vi "Main.vi"() -> ()   [LabVIEW 2020] (continued)
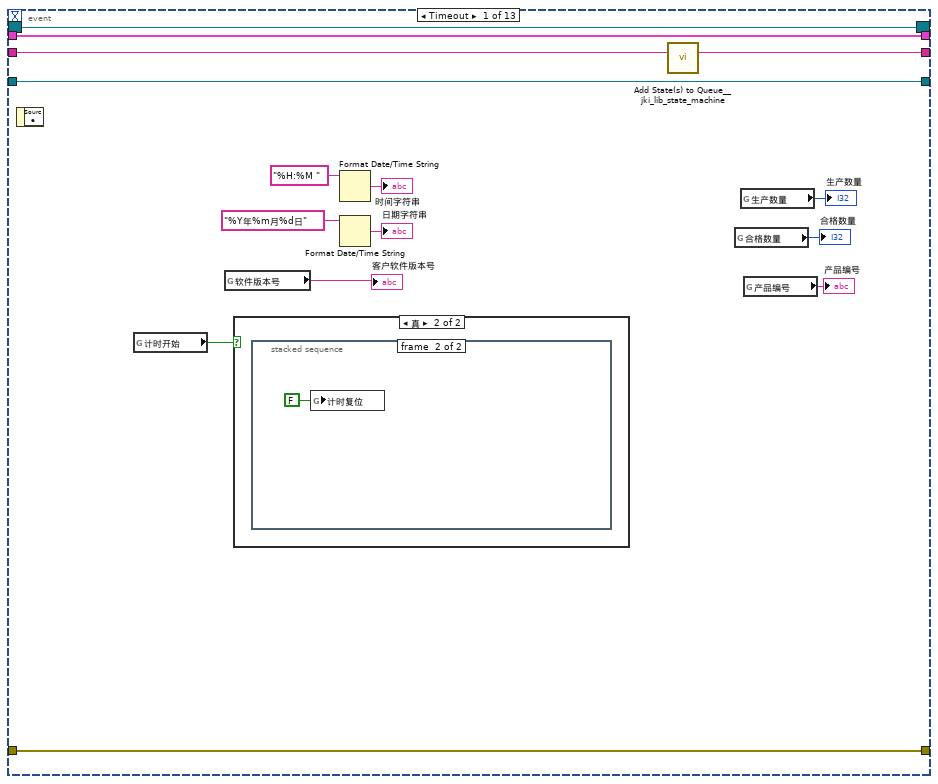
[diagram p2: hidden frame]
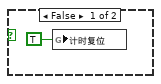
[diagram p3: hidden frame]
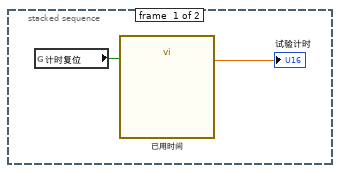
[diagram p4: hidden frame]
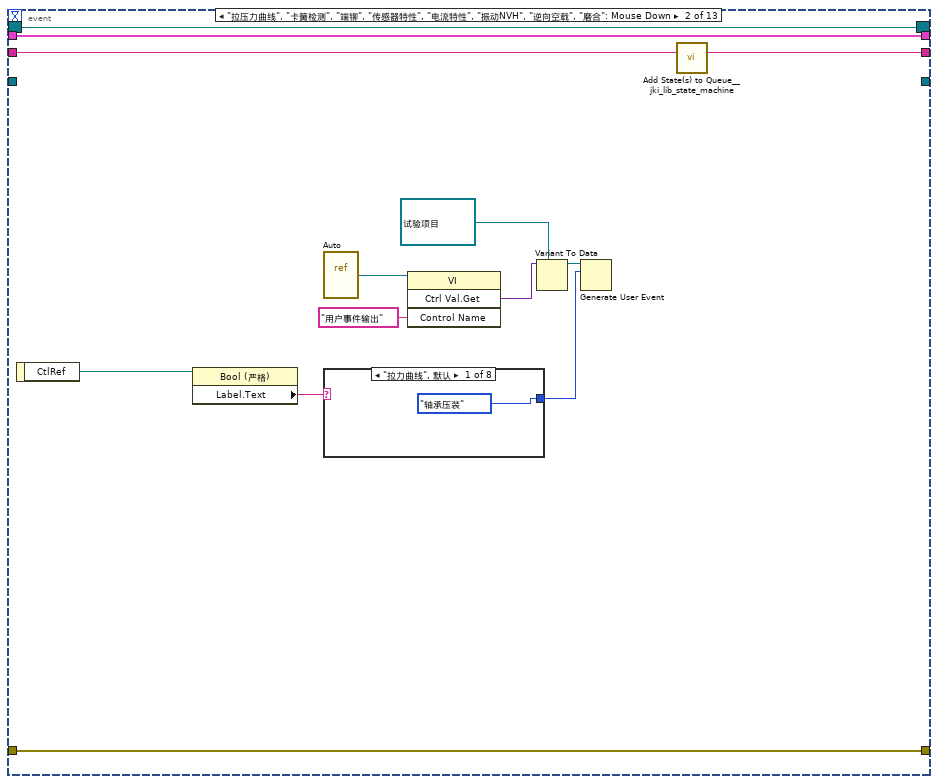
[diagram p5: hidden frame]
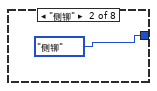
[diagram p6: hidden frame]
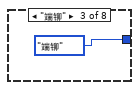
[diagram p7: hidden frame]
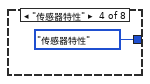
[diagram p8: hidden frame]
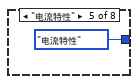
[diagram p9: hidden frame]
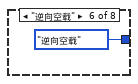
[diagram p10: hidden frame]
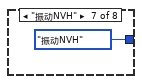
[diagram p11: hidden frame]
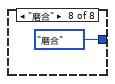
[diagram p12: hidden frame]
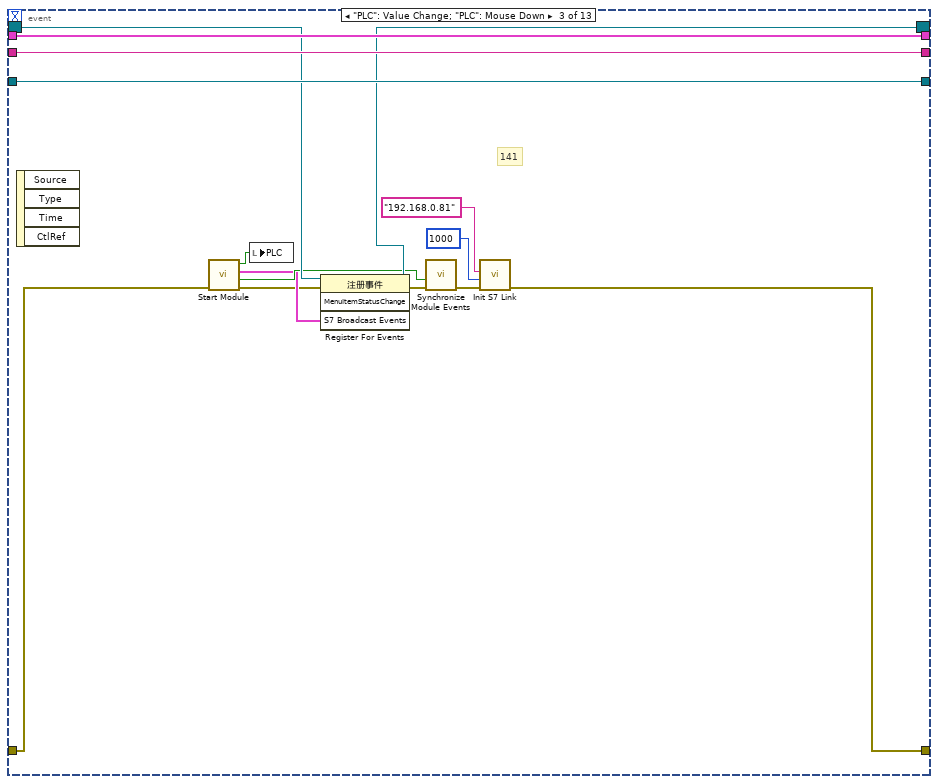
[diagram p13: hidden frame]
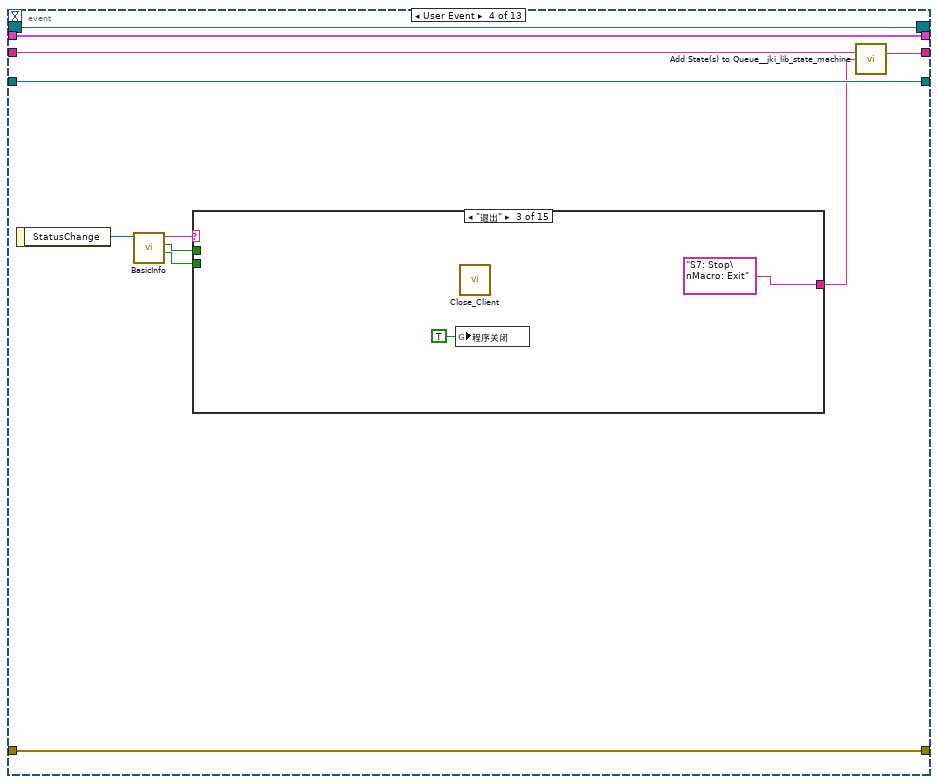
[diagram p14: hidden frame]
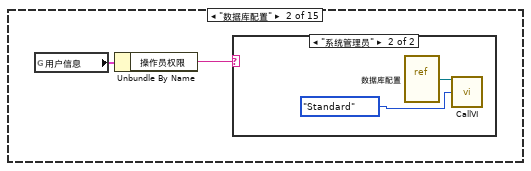
[diagram p16: hidden frame]
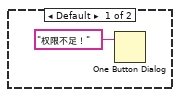
[diagram p17: hidden frame]
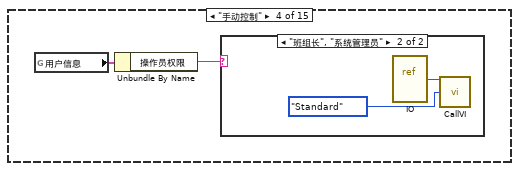
[diagram p18: hidden frame]
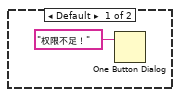
[diagram p19: hidden frame]
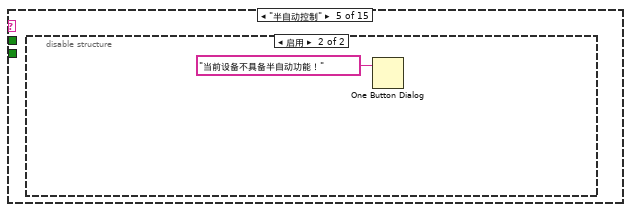
[diagram p20: hidden frame]
                    n120 = case shown="真" w200 {
                      frame False {
                      }
                      frame True {
                        n121 = vi-ref "Auto.vi"() -> (w204:refnum<vi>)
                        n122 = invoke class="VI" method="Ctrl Val.Set"(reference=w204, "Control Name"="STEP" ("控件名"), "Value"="退出自动" ("控件名")) -> ()  [unwired: 2 in, 5 out]
                      }
                    }
                  }
                }
              }
              frame Enabled {
              }
            }
            n123 = call <vilib>:"Add State(s) to Queue__jki_lib_state_machine.vi"("State(s) in (\"\")"=w190) -> ("States Out"=w191:string)  [unwired: 14 in]
          }
          event "错误": Mouse Down {
            n124 = event-data() -> ()  [unwired: 1 in, 8 out]
            n125 = vi-ref "报警信息.vi"() -> (w207:refnum<vi>)
            n126 = call "CallVI.vi"("VI引用"=w207, "状态"=T4."Standard") -> ()  [unwired: 12 in, 2 out]
            n127 = call <vilib>:"Add State(s) to Queue__jki_lib_state_machine.vi"("State(s) in (\"\")"=w209) -> ("States Out"=w210:string)  [unwired: 14 in]
          }
          event Panel Close? {
            n128 = event-data() -> ()  [unwired: 1 in, 1 out]
            n129 = global write "Global.vi" "程序关闭"(TRUE ("程序关闭")) -> ()
            n130 = call <vilib>:"Add State(s) to Queue__jki_lib_state_machine.vi"("State(s) in Front (\"\")"="S7: Stop\nMacro: Exit", "State(s) in (\"\")"=w219) -> ("States Out"=w218:string)  [unwired: 13 in]
            n131 = event-data("Discard?"=TRUE) -> ()  [unwired: 1 in, 1 out]
          }
          event "更换产品": Value Change {
            n132 = event-data() -> ("NewVal"=w221:refnum<vi>)  [unwired: 1 in, 5 out]
            n133 = stacked-sequence {
              tunnel: w221 -> [w226]
              frame #0 {
                n134 = stacked-sequence {
                  tunnel: w226 -> [w234 _]
                  frame #0 {
                    n135 = disable-structure shown="禁用" {
                      disable-tunnel: w234 -> [w236 _]
                      frame Disabled {
                        n136 = control-ref of="子面板"() -> (w235:refnum<vi>)
                        n137 = call "Call_SubPanal.vi"("VI引用句柄"=w236, "SubPnl引用句柄"=w235) -> ()  [unwired: 9 in, 1 out]
                      }
                      frame Enabled {
                      }
                    }
                    n138 = vi-ref "Auto.vi"() -> (w233:refnum<vi>)
                    n139 = invoke class="VI" method="Ctrl Val.Get"(reference=w233, "Control Name"="产品变更_Event" ("控件名")) -> ("Get Control Value Variant"=w231:variant)  [unwired: 2 in, 3 out]
                    n140 = global read "Global.vi" "产品型号"() -> (w228:string)
                    n141 = Variant To Data(type=refnum<user-event> refnum ("产品变更_Event"), Variant=w231) -> (data=w229:refnum<user-event>, error out=w227:errorcluster)  [unwired: 1 in]
                    n142 = Generate User Event(user event=w229, event data cluster=w228, error in=w227) -> ()  [unwired: 1 in, 2 out]
                    n143 = local write "产品型号"(w228) -> ()
                  }
                  frame #1 {
                    n144 = disable-structure shown="禁用" {
                      frame Disabled {
                        n145 = control-ref of="拉压力曲线"() -> (w238:refnum<vi>)
                        n146 = control-ref of="卡簧检测"() -> (w237:refnum<vi>)
                        n147 = global read "Global.vi" "试验项目"() -> (w241:bool[])
                        n148 = Build Array(w238, w237) -> (w240:refnum<vi>[])
                        n149 = for {
                          tunnel: w240 -> [w245] mode=indexing
                          tunnel: w241 -> [w246] mode=indexing
                          shift-right: [w242] -> _
                          shift-left: 2000 -> [w243]
                          i -> [w244]
                          n150 = case shown="真" w246 {
                            tunnel: w245 -> [w247 w255]
                            tunnel: w244 -> [_ _]
                            tunnel: w243 -> [w249 w252]
                            tunnel: [w249 w250] -> w242
                            frame False {
                              n151 = property class="Bool (严格)"(reference=w247, "Top"=2000) -> ()  [unwired: 1 in, 2 out]
                            }
                            frame True {
                              n152 = Add(x=w252, y=135) -> (x+y=w250:i32)
                              n153 = Bundle(w250, 1235) -> (w253:cluster{i32, i32})  [unwired: 1 in]
                              n154 = property class="Bool (严格)"(reference=w255, "Position"=w253) -> ()  [unwired: 1 in, 2 out]
                            }
                          }
                        }
                      }
                      frame Enabled {
                      }
                    }
                  }
                }
              }
            }
            n155 = call <vilib>:"Add State(s) to Queue__jki_lib_state_machine.vi"("State(s) in (\"\")"=w222) -> ("States Out"=w223:string)  [unwired: 14 in]
          }
          event "Andon": Value Change {
            n156 = event-data() -> ("NewVal"=w260:enum32{"未选择", "缺料报警", "质量报警", "故障报警"})  [unwired: 1 in]
            n157 = case shown="\"未选择\", 默认" w260 {
              tunnel: [enum16{"设备离线", "设备正常", "设备缺料", "设备故障", "质量报警"}."设备正常" ("设备状态") enum16{"设备离线", "设备正常", "设备缺料", "设备故障", "质量报警"}."设备缺料" ("设备状态") enum16{"设备离线", "设备正常", "设备缺料", "设备故障", "质量报警"}."质量报警" ("设备状态") enum16{"设备离线", "设备正常", "设备缺料", "设备故障", "质量报警"}."设备故障" ("设备状态")] -> w258
              frame "未选择", Default {
              }
              frame "缺料报警" {
              }
              frame "质量报警" {
              }
              frame "故障报警" {
              }
            }
            n158 = local read "userName"() -> (w257:string)
            n159 = Bundle By Name(cluster=T5 {"设备名称"="滑移力检测", "操作人员"="", "设备状态"=enum."设备离线", "附加信息"=""} ("设备信息"), "操作人员"=w257, "设备状态"=w258) -> (w256:T5)
            n160 = call "Change_Client.vi"("设备信息"=w256) -> ()  [unwired: 10 in, 1 out]
          }
        }
      }
      frame "---------- Core ----------" {
        n161 = call <vilib>:"Add State(s) to Queue__jki_lib_state_machine.vi"("State(s) in (\"\")"=w274) -> ("States Out"=w273:string)  [unwired: 14 in]
      }
      frame Default {
        w286 = 42 items=["No error", "Argument error", "Memory is full", "Out of zone", "End of file", "File already open", "Generic file I/O error", "File not found", "File permission error", "Disk is full", "Duplicate path", "Too many files open", "System feature not enabled", "Resource file not found", "Cannot add resource", "Resource not found", "Image not found", "Image memory error", "Pen does not exist", "Config type invalid", "Config token not found", "Config parse error", "Config memory error", "Bad external code format", "Bad external code offset", "External code not present", "Null window", "Destroy window error", "Null menu", "Print aborted", "Bad print record", "Print driver error", "Windows error during printing", "Memory error during printing", "Print dialog error", "Generic print error", "Invalid device refnum", "Device not found", "Device parameter error", "Device unit error", "Cannot open device", "Device call aborted", "Generic error", "Cancelled by user", "Object ID too low", "Object ID too high", "Object not in heap", "Unknown heap", "Unknown object (invalid DefProc)", "Unknown object (DefProc not in table)", "Message out of range", "Invalid (null) method", "Unknown message", "Manager call not supported", "Bad address", "Network operation in progress", "Network operation timed out", "Connection is busy", "Network attribute not supported", "Network error", "Address in use", "System out of memory", "Connection aborted", "Connection refused", "Not connected", "Already connected", "Connection closed", "Initialization error (interapplication manager)", "Bad occurrence", "Wait on unbound occurrence handler", "Occurrence queue overflow", "Datalog type conflict", "Unused", "Unrecognized type (interapplication manager)", "Memory corrupt", "Failed to make temporary DLL", "Old CIN version", "Drag socket not found", "Failed to load drop-object", "Failed to register OLE object", "Failed to release OLE object", "Format specifier type mismatch", "Unknown format specifier", "Too few format specifiers", "Too many format specifiers", "Scan failed", "Newer CIN version", "Error converting to variant", "Runtime menu error", "Password tampered", "Variant attribute not found", "Incompatible variant data type", "Event data is not available", "Event Store is not present", "Occurrence is not found", "Event Queue is not created", "Event info is not available", "Refnum passed is NULL", "Error retrieving Class GUID", "Error retrieving CoClass GUID", "Error retrieving TypeLib GUID.", "Bad built application magic bytes.", "Specific driver is different from the specific driver associated with the Logical Name.", "There is no session opened to the class driver.", "Max Error", "MAX - Error with config objects", "MAX - Error loading configuration", "MAX - Group not supported"]
        # "Current State"
        n162 = Format Into String(format string="Software Exception: Unhandled State \"%s\"." ("message"), error in=w282, w277) -> (resulting string=w285:string, error out=w284:errorcluster)  [unwired: 1 in]
        n163 = call <vilib>:"Error Cluster From Error Code.vi"("show call chain? (False)"=TRUE, "error in (no error)"=w284, "error message (\"\")"=w285, "error code (0)"=w286) -> ("error out"=w283:errorcluster)  [unwired: 5 in]
        n164 = call <vilib>:"Add State(s) to Queue__jki_lib_state_machine.vi"("State(s) in (\"\")"=w281) -> ("States Out"=w280:string)  [unwired: 14 in]
      }
      frame "Initialize Core Data" {
        # "originally closed?"
        # "exe?"
        n165 = property class="VI"() -> ("Front Panel.Open"=w297:bool)  [unwired: 2 in, 2 out]
        n166 = property class="App"() -> ("App.Kind"=w296:T6)  [unwired: 2 in, 2 out]
        n167 = control-ref of="Current VI Reference"() -> (w290:refnum<vi>)
        n168 = Not(x=w297) -> (.not. x?=w294:bool)
        n169 = Equal?(x=w296, y=T6."Run Time System" ("Application:Kind")) -> (x = y?=w293:bool)
        n170 = Or(x=w294, y=w293) -> (x .or. y?=w291:bool)
        n171 = Bundle By Name(cluster=w292, "Core.Current VI Reference"=w290, "Core.Close Panel on Exit?"=w291) -> (w299:T8)
        n172 = call <vilib>:"Add State(s) to Queue__jki_lib_state_machine.vi"("State(s) in (\"\")"=w301) -> ("States Out"=w300:string)  [unwired: 14 in]
      }
      frame "Error Handler" {
        n173 = call <vilib>:"General Error Handler.vi"("error in (no error)"=w305) -> ()  [unwired: 10 in, 5 out]
        n174 = call <vilib>:"Add State(s) to Queue__jki_lib_state_machine.vi"("State(s) in Front (\"\")"="/* Post Error States", "State(s) in (\"\")"=w309) -> ("States Out"=w308:string)  [unwired: 13 in]
      }
      frame "Exit" {
        n175 = call <vilib>:"Add State(s) to Queue__jki_lib_state_machine.vi"("State(s) in (\"\")"=w316) -> ("States Out"=w315:string)  [unwired: 14 in]
        n176 = Quit LabVIEW() -> ()  [unwired: 1 in]
      }
      frame "--------- Library --------" {
        n177 = call <vilib>:"Add State(s) to Queue__jki_lib_state_machine.vi"("State(s) in (\"\")"=w322) -> ("States Out"=w321:string)  [unwired: 14 in]
      }
      frame "S7: Initialize" {
        n178 = property on="PLC" class="Bool (严格)"("Val(Sgnl)"=FALSE ("值(信号)")) -> ()  [unwired: 2 in, 2 out]
      }
      frame "S7: Stop" {
        n179 = call "Stop Module.vi"("error in (no error)"=w331) -> ("error out"=w330:errorcluster)  [unwired: 10 in]
        n180 = call <vilib>:"Add State(s) to Queue__jki_lib_state_machine.vi"("State(s) in (\"\")"=w332) -> ("States Out"=w333:string)  [unwired: 14 in]
      }
      frame "CAN: Start" {
        n181 = call <vilib>:"Add State(s) to Queue__jki_lib_state_machine.vi"("State(s) in (\"\")"=w338) -> ("States Out"=w339:string)  [unwired: 14 in]
      }
      frame "CAN: Stop" {
        n182 = call <vilib>:"Add State(s) to Queue__jki_lib_state_machine.vi"("State(s) in (\"\")"=w344) -> ("States Out"=w345:string)  [unwired: 14 in]
      }
      frame "---------- Data ----------" {
        n183 = call <vilib>:"Add State(s) to Queue__jki_lib_state_machine.vi"("State(s) in (\"\")"=w353) -> ("States Out"=w352:string)  [unwired: 14 in]
      }
      frame "Data: Initialize" {
        w358 = T9 {"Current VI Reference"=refnum, "Close Panel on Exit?"=FALSE}  # Core
        w360 = TRUE  # Your Boolean data
        w359 = ""  # Your string data
        n184 = global write "Global.vi" "程序关闭"(FALSE ("程序关闭")) -> ()
        n185 = global write "Global.vi" "计时开始"(FALSE ("计时结束")) -> ()
        n186 = Bundle("Core"=w358, "Your Boolean data"=w360, "Your string data"=w359) -> (w362:T8)  [unwired: 1 in]
        n187 = call <vilib>:"Add State(s) to Queue__jki_lib_state_machine.vi"("State(s) in (\"\")"=w364) -> ("States Out"=w363:string)  [unwired: 14 in]
      }
      frame "Data: Cleanup" {
        n188 = Unbundle By Name(w367) -> ("Core.Current VI Reference"=w370:refnum<vi>)
        n189 = Close Reference(reference=w370, error in (no error)=w369) -> (error out=w368:errorcluster)
        n190 = call <vilib>:"Add State(s) to Queue__jki_lib_state_machine.vi"("State(s) in (\"\")"=w372) -> ("States Out"=w371:string)  [unwired: 14 in]
      }
      frame "---------- UI ----------" {
        # "Do not put any code in this frame.\n(It is a separator no-op. You can make a copy of this frame to create a new UI frame)"
        n191 = call <vilib>:"Add State(s) to Queue__jki_lib_state_machine.vi"("State(s) in (\"\")"=w378) -> ("States Out"=w377:string)  [unwired: 14 in]
      }
      frame "UI: Initialize" {
        n192 = disable-structure shown="启用" {
          disable-tunnel: [w388 _] -> w382
          disable-tunnel: w379 -> [w386 _]
          frame Enabled {
            n193 = vi-ref "Auto.vi"() -> (w387:refnum<vi>)
            n194 = invoke on="子面板" class="SubPnl" method="Insert VI"(error in=w386, "VI Ref"=w387) -> (error out=w391:errorcluster)  [unwired: 2 in, 3 out]
            n195 = invoke class="VI" method="Run VI"(reference=w387, error in=w391, "Wait until done"=FALSE ("结束前等待"), "Auto Dispose Ref"=TRUE ("自动销毁引用")) -> (error out=w388:errorcluster)  [unwired: 1 in, 4 out]
          }
          frame Disabled {
            n196 = vi-ref "Auto.vi"() -> (w393:refnum<vi>)
            n197 = call "CallVI.vi"("VI引用"=w393, "状态"=T4."Maximized") -> ()  [unwired: 12 in, 2 out]
          }
        }
        n198 = call <vilib>:"Add State(s) to Queue__jki_lib_state_machine.vi"("State(s) in (\"\")"=w385) -> ("States Out"=w384:string)  [unwired: 14 in]
      }
      frame "UI: Init" {
        n199 = stacked-sequence {
          tunnel: w395 -> [_ _ _ _]
          frame #0 {
            n200 = global write "Global.vi" "程序关闭"(FALSE ("程序关闭")) -> ()
            n201 = control-ref of="拉压力曲线"() -> (w407:refnum<vi>)
            n202 = control-ref of="电流特性"() -> (w404:refnum<vi>)
            n203 = control-ref of="端铆"() -> (w405:refnum<vi>)
            n204 = control-ref of="卡簧检测"() -> (w406:refnum<vi>)
            n205 = global write "A180648.vi" "LED-轴承压装"(w407) -> ()
            n206 = global write "A180648.vi" "LED-电流特性"(w404) -> ()
            n207 = global write "A180648.vi" "LED-侧铆"(w406) -> ()
            n208 = global write "A180648.vi" "LED-端铆"(w405) -> ()
            n209 = control-ref of="逆向空载"() -> (w403:refnum<vi>)
            n210 = control-ref of="振动NVH"() -> (w401:refnum<vi>)
            n211 = control-ref of="传感器特性"() -> (w402:refnum<vi>)
            n212 = control-ref of="磨合"() -> (w400:refnum<vi>)
            n213 = global write "A180648.vi" "LED-传感器特性"(w402) -> ()
            n214 = global write "A180648.vi" "LED-逆向空载"(w403) -> ()
            n215 = global write "A180648.vi" "LED-振动NVH"(w401) -> ()
            n216 = global write "A180648.vi" "LED-磨合"(w400) -> ()
          }
          frame #1 {
            w415 = 0
            n217 = shared-variable "我的电脑\\Global.lvlib\\总成追溯码"("   " ("工位追溯码")) -> ()  [unwired: 1 in, 1 out]
            n218 = global write "Global.vi" "生产数量"(w415) -> ()
            n219 = global write "Global.vi" "合格数量"(w415) -> ()
            n220 = global read "Global.vi" "用户信息"() -> (w412:T10)
            n221 = global read "Global.vi" "联机模式"() -> (w409:enum16{"单机", "追溯"})
            n222 = Unbundle By Name(w412) -> ("用户名"=→"userName":string, "用户权限"=→"userStatus":string)
            n223 = case shown="\"追溯\"" w409 {
              tunnel: ["联网" ("connectionMode") "单机" ("connectionMode")] -> w416
              frame "追溯" {
              }
              frame "单机", Default {
              }
            }
            "connectionMode" <- w416
            "产品型号" <- "" ("产品型号")
          }
          frame #2 {
            n224 = control-ref of="提示信息"() -> (w421:refnum<vi>)
            n225 = control-ref of="自动"() -> (w422:refnum<vi>)
            n226 = control-ref of="错误"() -> (w423:refnum<vi>)
            n227 = control-ref of="Result"() -> (w424:refnum<vi>)
            n228 = control-ref of="更换产品"() -> (w420:refnum<vi>)
            n229 = global write "Global.vi" "提示信息"(w421) -> ()
            n230 = global write "Global.vi" "程序自动"(w422) -> ()
            n231 = global write "Global.vi" "报警图标"(w423) -> ()
            n232 = global write "Global.vi" "Result"(w424) -> ()
            n233 = global write "Global.vi" "更换产品"(w420) -> ()
            n234 = control-ref of="状态"() -> (w419:refnum<vi>)
            n235 = global write "Global.vi" "状态"(w419) -> ()
          }
          frame #3 {
            n236 = global read "Global.vi" "Result"() -> (w427:refnum<vi>)
            n237 = property class="Tbl"(reference=w427, "Row Headers[]"=string[] [], "Value"=string[][] []) -> ()  [unwired: 1 in, 2 out]
            n238 = call "Start_Client.vi"() -> ()  [unwired: 12 in]
          }
        }
        n239 = call <vilib>:"Add State(s) to Queue__jki_lib_state_machine.vi"("State(s) in (\"\")"=w399) -> ("States Out"=w398:string)  [unwired: 14 in]
      }
      frame "UI: Config" {
        n240 = vi-ref "Config.vi"() -> (w430:refnum<vi>)
        n241 = call "CallVI.vi"("VI引用"=w430, "状态"=T4."Standard") -> ()  [unwired: 12 in, 2 out]
        n242 = call <vilib>:"Add State(s) to Queue__jki_lib_state_machine.vi"("State(s) in (\"\")"=w435) -> ("States Out"=w434:string)  [unwired: 14 in]
      }
      frame "UI: Cursor Set" {
        # "Argument"
        n243 = case shown="\"Idle\", 默认" w438 {
          tunnel: w440 -> [w445 w447]
          tunnel: [w444 w446] -> w439
          frame "Idle", Default {
            n244 = call <vilib>:"Unset Busy.vi"("error in (no error)"=w445) -> ("error out"=w444:errorcluster)  [unwired: 10 in]
          }
          frame "Busy" {
            n245 = call <vilib>:"Set Busy.vi"("error in (no error)"=w447) -> ("error out"=w446:errorcluster)  [unwired: 9 in, 1 out]
          }
        }
        n246 = call <vilib>:"Add State(s) to Queue__jki_lib_state_machine.vi"("State(s) in (\"\")"=w443) -> ("States Out"=w442:string)  [unwired: 14 in]
      }
      frame "UI: Front Panel State" {
        # "Argument"
        n247 = Unbundle By Name(w452) -> ("Core.Current VI Reference"=w451:refnum<vi>)
        n248 = case shown="\"Close\"" w450 {
          tunnel: w454 -> [w460 w473]
          tunnel: [w462 w474] -> w453
          tunnel: w451 -> [w461 w471]
          frame "Open", Default {
            n249 = property class="VI"(reference=w461, error in=w460) -> (reference out=w458:refnum<vi>, error out=w459:errorcluster, "Front Panel.Open"=w457:bool)
            n250 = case shown="假" w457 {
              tunnel: [w465 w468] -> w462
              tunnel: w459 -> [w464 w468]
              tunnel: w458 -> [w463 _]
              frame False {
                n251 = invoke class="VI" method="FP.Open"(reference=w463, error in=w464, "Activate"=TRUE, "State"=T4."Standard") -> (error out=w465:errorcluster)  [unwired: 1 in, 4 out]
              }
              frame True {
              }
            }
          }
          frame "Close" {
            n252 = property class="VI"(reference=w471, error in=w473) -> (reference out=w470:refnum<vi>, error out=w472:errorcluster, "Front Panel.Open"=w469:bool)
            n253 = case shown="真" w469 {
              tunnel: [w475 w478] -> w474
              tunnel: w472 -> [w475 w477]
              tunnel: w470 -> [_ w476]
              frame False {
              }
              frame True {
                n254 = invoke class="VI" method="FP.Close"(reference=w476, error in=w477) -> (error out=w478:errorcluster)  [unwired: 1 in, 2 out]
              }
            }
          }
        }
        n255 = call <vilib>:"Add State(s) to Queue__jki_lib_state_machine.vi"("State(s) in (\"\")"=w456) -> ("States Out"=w455:string)  [unwired: 14 in]
      }
      frame "---------- Macro ----------" {
        n256 = call <vilib>:"Add State(s) to Queue__jki_lib_state_machine.vi"("State(s) in (\"\")"=w484) -> ("States Out"=w483:string)  [unwired: 14 in]
      }
      frame "Macro: Initialize" {
        n257 = call <vilib>:"Add State(s) to Queue__jki_lib_state_machine.vi"("State(s) in Front (\"\")"="Data: Initialize\nInitialize Core Data\nS7: Initialize\nIdle\nUI: Init\nUI: Front Panel State >> Open\nUI: Initialize\nUI: Config", "State(s) in (\"\")"=w491) -> ("States Out"=w490:string)  [unwired: 13 in]
      }
      frame "Macro: Exit" {
        n258 = Unbundle By Name(w500) -> ("Core.Close Panel on Exit?"=w499:bool)
        n259 = Select(t="UI: Front Panel State >> Close", s=w499, f="") -> (s? t:f=w496:string)
        n260 = call <vilib>:"Add State(s) to Queue__jki_lib_state_machine.vi"("State(s) in (\"\")"=w496, "State(s) at Back (\"\")"="Data: Cleanup\nExit") -> ("States Out"=w494:string)  [unwired: 13 in]
        n261 = call <vilib>:"Add State(s) to Queue__jki_lib_state_machine.vi"("State(s) in Front (\"\")"=w494, "State(s) in (\"\")"=w503) -> ("States Out"=w502:string)  [unwired: 13 in]
      }
    }
  }
  n262 = call-dynamic "Cleanup.vi"("MenuStrip in"=w6) -> ()  [unwired: 10 in, 1 out]
